vi "Dresden R2R Sputter 03.02.2018 IY24.vi"() -> ()   [LabVIEW 2009] (continued)
                                }
                                }
                                frame #1 {
                                n17381 = local read "Semi"() -> (w25829:bool)
                                n17382 = case shown="False" w25829 {
                                frame #0 {
                                n17383 = local write "Ch2_PV13"(TRUE ("P03")) -> ()
                                n17384 = Wait Until Next ms Multiple(millisecond multiple=u32 1000) -> ()  [unwired: 1 out]
                                }
                                frame #1 {
                                }
                                }
                                }
                                }
                              }
                              frame #1 {
                              }
                            }
                          }
                          frame #8 {
                            # "OPEN PC-BV"
                            n17385 = local read "Semi"() -> (w25832:bool)
                            n17386 = case shown="False" w25832 {
                              frame #0 {
                                n17387 = stacked-sequence {
                                frame #0 {
                                n17388 = local read "Semi"() -> (w25833:bool)
                                n17389 = case shown="False" w25833 {
                                frame #0 {
                                n17390 = stacked-sequence {
                                frame #0 {
                                n17391 = local read "Semi"() -> (w25834:bool)
                                n17392 = case shown="False" w25834 {
                                frame #0 {
                                n17393 = local write "Pc_bv2_auto_open"(TRUE ("Tp1_auto_start")) -> ()
                                }
                                frame #1 {
                                }
                                }
                                }
                                frame #1 {
                                n17394 = local read "Semi"() -> (w25836:bool)
                                n17395 = case shown="False" w25836 {
                                frame #0 {
                                n17396 = Wait (ms)(milliseconds to wait=u32 1000) -> ()  [unwired: 1 out]
                                }
                                frame #1 {
                                }
                                }
                                }
                                frame #2 {
                                n17397 = local read "Semi"() -> (w25838:bool)
                                n17398 = case shown="False" w25838 {
                                frame #0 {
                                n17399 = while {
                                i -> [w25844]
                                stop <- w25840 stop-if-true
                                n17400 = local read "Pc_bv_opened_ch2"() -> (w25842:bool)
                                n17401 = Greater?(x=w25844, y=120) -> (0:w25843:bool)
                                n17402 = local read "Semi"() -> (w25841:bool)
                                n17403 = Compound Arithmetic op=OR(w25841, w25842, w25843) -> (w25840:bool)
                                n17404 = Wait (ms)(milliseconds to wait=u32 500) -> ()  [unwired: 1 out]
                                }
                                }
                                frame #1 {
                                }
                                }
                                }
                                frame #3 {
                                n17405 = local read "Semi"() -> (w25846:bool)
                                n17406 = case shown="False" w25846 {
                                frame #0 {
                                n17407 = local read "Pc_bv_opened_ch2"() -> (w25847:bool)
                                n17408 = case shown="False" w25847 {
                                frame #0 {
                                n17409 = local write "Pc_bv2_auto_open"(TRUE ("Pc_bv1_auto_open")) -> ()
                                }
                                frame #1 {
                                }
                                }
                                }
                                frame #1 {
                                }
                                }
                                }
                                frame #4 {
                                n17410 = local read "Semi"() -> (w25849:bool)
                                n17411 = case shown="False" w25849 {
                                frame #0 {
                                n17412 = local read "Pc_bv_opened_ch2"() -> (w25850:bool)
                                n17413 = case shown="False" w25850 {
                                frame #0 {
                                n17414 = Wait (ms)(milliseconds to wait=u32 1000) -> ()  [unwired: 1 out]
                                }
                                frame #1 {
                                }
                                }
                                }
                                frame #1 {
                                }
                                }
                                }
                                frame #5 {
                                n17415 = local read "Semi"() -> (w25852:bool)
                                n17416 = case shown="False" w25852 {
                                frame #0 {
                                n17417 = while {
                                i -> [w25858]
                                stop <- w25854 stop-if-true
                                n17418 = local read "Pc_bv_opened_ch2"() -> (w25856:bool)
                                n17419 = Greater?(x=w25858, y=120) -> (0:w25857:bool)
                                n17420 = local read "Semi"() -> (w25855:bool)
                                n17421 = Compound Arithmetic op=OR(w25855, w25856, w25857) -> (w25854:bool)
                                n17422 = Wait (ms)(milliseconds to wait=u32 500) -> ()  [unwired: 1 out]
                                }
                                }
                                frame #1 {
                                }
                                }
                                }
                                frame #6 {
                                n17423 = local read "Semi"() -> (w25860:bool)
                                n17424 = case shown="False" w25860 {
                                frame #0 {
                                n17425 = local read "Pc_bv_opened_ch2"() -> (w25861:bool)
                                n17426 = case shown="False" w25861 {
                                frame #0 {
                                n17427 = local write "Error Message"("Start up process  cancelled\nbecause  PC-BV not opened.\nPlease check PC-BV2 connections." ("Error Message")) -> ()
                                n17428 = Wait (ms)(milliseconds to wait=u32 1000) -> ()  [unwired: 1 out]
                                }
                                frame #1 {
                                }
                                }
                                }
                                frame #1 {
                                }
                                }
                                }
                                }
                                }
                                frame #1 {
                                }
                                }
                                }
                                frame #1 {
                                n17429 = local read "Semi"() -> (w25864:bool)
                                n17430 = case shown="False" w25864 {
                                frame #0 {
                                n17431 = local write "Ch2_PV14"(TRUE ("P03")) -> ()
                                n17432 = Wait Until Next ms Multiple(millisecond multiple=u32 1000) -> ()  [unwired: 1 out]
                                }
                                frame #1 {
                                }
                                }
                                }
                                }
                              }
                              frame #1 {
                              }
                            }
                          }
                          frame #9 {
                            # "OPEN/CLOSE TRNS GV-BP2"
                            n17433 = local read "Semi"() -> (w25867:bool)
                            n17434 = case shown="False" w25867 {
                              frame #0 {
                                n17435 = stacked-sequence {
                                frame #0 {
                                n17436 = local read "Semi"() -> (w25868:bool)
                                n17437 = case shown="False" w25868 {
                                frame #0 {
                                n17438 = while {
                                i -> [w25877]
                                stop <- w25872 stop-if-true
                                n17439 = Greater?(x=w25877, y=50) -> (0:w25875:bool)
                                n17440 = case shown="True" w25875 {
                                frame #0 {
                                }
                                frame #1 {
                                n17441 = local read "Ch3_pressure"() -> (w25891:dbl)
                                n17442 = Less?(x=w25891, y=1) -> (x < y?=w25890:bool)
                                n17443 = case shown="True" w25890 {
                                frame #0 {
                                n17444 = local write "Error Message"("Start up process  cancelled\nbecause  Trns GV-BP2 not closed.\nPlease check \nTrns GV-BP2 connections." ("Error Message")) -> ()
                                }
                                frame #1 {
                                n17445 = local write "Error Message"("Start up process  cancelled\nbecause  Trns GV-BP2 not opened.\nPlease check \nTrns GV-BP2 connections." ("Error Message")) -> ()
                                }
                                }
                                n17446 = local write "Semi"(TRUE ("Semi")) -> ()
                                }
                                }
                                n17447 = local read "Ch3_pressure"() -> (w25871:dbl)
                                n17448 = Less?(x=w25871, y=1) -> (x < y?=w25869:bool)
                                n17449 = case shown="False" w25869 {
                                tunnel: [w25879 w25885] -> w25874
                                frame #0 {
                                n17450 = local read "Ch2_trns_gv_bp2_di"() -> (w25878:bool)
                                n17451 = case shown="True" w25878 {
                                tunnel: [TRUE FALSE] -> w25879
                                frame #0 {
                                }
                                frame #1 {
                                n17452 = local write "Ch2_trns_gv_bp2_do"(FALSE ("Ch1_Tp_bv_do")) -> ()
                                n17453 = Wait Until Next ms Multiple(millisecond multiple=u32 200) -> ()  [unwired: 1 out]
                                }
                                }
                                }
                                frame #1 {
                                n17454 = local read "Ch2_trns_gv_bp2_di"() -> (w25884:bool)
                                n17455 = case shown="False" w25884 {
                                tunnel: [FALSE TRUE] -> w25885
                                frame #0 {
                                n17456 = local write "Ch2_trns_gv_bp2_do"(TRUE ("Ch1_Tp_bv_do")) -> ()
                                n17457 = Wait Until Next ms Multiple(millisecond multiple=u32 200) -> ()  [unwired: 1 out]
                                }
                                frame #1 {
                                }
                                }
                                }
                                }
                                n17458 = local read "Semi"() -> (w25873:bool)
                                n17459 = Or(x=w25874, y=w25873) -> (x .or. y?=w25872:bool)
                                }
                                }
                                frame #1 {
                                }
                                }
                                }
                                frame #1 {
                                n17460 = local read "Semi"() -> (w25896:bool)
                                n17461 = case shown="False" w25896 {
                                frame #0 {
                                n17462 = local write "Ch2_PV15"(TRUE ("P03")) -> ()
                                n17463 = Wait Until Next ms Multiple(millisecond multiple=u32 1000) -> ()  [unwired: 1 out]
                                }
                                frame #1 {
                                }
                                }
                                }
                                }
                              }
                              frame #1 {
                              }
                            }
                          }
                          frame #10 {
                            # "OPEN/CLOSE TRNS GV-BP"
                            n17464 = local read "Semi"() -> (w25899:bool)
                            n17465 = case shown="False" w25899 {
                              frame #0 {
                                n17466 = stacked-sequence {
                                frame #0 {
                                n17467 = local read "Semi"() -> (w25900:bool)
                                n17468 = case shown="False" w25900 {
                                frame #0 {
                                n17469 = while {
                                i -> [w25909]
                                stop <- w25904 stop-if-true
                                n17470 = Greater?(x=w25909, y=50) -> (0:w25907:bool)
                                n17471 = case shown="True" w25907 {
                                frame #0 {
                                }
                                frame #1 {
                                n17472 = local read "Ch1_pressure"() -> (w25923:dbl)
                                n17473 = Less?(x=w25923, y=1) -> (x < y?=w25922:bool)
                                n17474 = case shown="True" w25922 {
                                frame #0 {
                                n17475 = local write "Error Message"("Start up process  cancelled\nbecause  Trns GV-BP2 not closed.\nPlease check \nTrns GV-BP2 connections." ("Error Message")) -> ()
                                }
                                frame #1 {
                                n17476 = local write "Error Message"("Start up process  cancelled\nbecause  Trns GV-BP not opened.\nPlease check \nTrns GV-BP connections." ("Error Message")) -> ()
                                }
                                }
                                n17477 = local write "Semi"(TRUE ("Semi")) -> ()
                                }
                                }
                                n17478 = local read "Ch1_pressure"() -> (w25903:dbl)
                                n17479 = Less?(x=w25903, y=1) -> (x < y?=w25901:bool)
                                n17480 = case shown="True" w25901 {
                                tunnel: [w25911 w25917] -> w25906
                                frame #0 {
                                n17481 = local read "Ch2_trns_gv_bp_di"() -> (w25910:bool)
                                n17482 = case shown="True" w25910 {
                                tunnel: [TRUE FALSE] -> w25911
                                frame #0 {
                                }
                                frame #1 {
                                n17483 = local write "Ch2_trns_gv_bp_do"(FALSE ("Ch1_Tp_bv_do")) -> ()
                                n17484 = Wait Until Next ms Multiple(millisecond multiple=u32 200) -> ()  [unwired: 1 out]
                                }
                                }
                                }
                                frame #1 {
                                n17485 = local read "Ch2_trns_gv_bp_di"() -> (w25916:bool)
                                n17486 = case shown="False" w25916 {
                                tunnel: [FALSE TRUE] -> w25917
                                frame #0 {
                                n17487 = local write "Ch2_trns_gv_bp_do"(TRUE ("Ch1_Tp_bv_do")) -> ()
                                n17488 = Wait Until Next ms Multiple(millisecond multiple=u32 200) -> ()  [unwired: 1 out]
                                }
                                frame #1 {
                                }
                                }
                                }
                                }
                                n17489 = local read "Semi"() -> (w25905:bool)
                                n17490 = Or(x=w25906, y=w25905) -> (x .or. y?=w25904:bool)
                                }
                                }
                                frame #1 {
                                }
                                }
                                }
                                frame #1 {
                                n17491 = local read "Semi"() -> (w25928:bool)
                                n17492 = case shown="False" w25928 {
                                frame #0 {
                                n17493 = local write "Ch2_PV16"(TRUE ("P03")) -> ()
                                n17494 = Wait Until Next ms Multiple(millisecond multiple=u32 1000) -> ()  [unwired: 1 out]
                                }
                                frame #1 {
                                }
                                }
                                }
                                }
                              }
                              frame #1 {
                              }
                            }
                          }
                          frame #11 {
                            # "CHECK CH-PRESSURE"
                            n17495 = local read "Semi"() -> (w25931:bool)
                            n17496 = case shown="False" w25931 {
                              frame #0 {
                                n17497 = stacked-sequence {
                                frame #0 {
                                n17498 = local read "Semi"() -> (w25932:bool)
                                n17499 = case shown="False" w25932 {
                                frame #0 {
                                n17500 = while {
                                i -> [w25941]
                                stop <- w25936 stop-if-true
                                n17501 = Greater?(x=w25941, y=600) -> (0:w25939:bool)
                                n17502 = case shown="True" w25939 {
                                frame #0 {
                                }
                                frame #1 {
                                n17503 = local write "Semi"(TRUE ("Semi")) -> ()
                                n17504 = local write "Error Message"("Start up process was cancelled.\nPlease check chamber \nvacuum connections." ("Error Message")) -> ()
                                }
                                }
                                n17505 = local read "Ch2_pressure"() -> (w25935:dbl)
                                n17506 = Less?(x=w25935, y=0.9) -> (x < y?=w25933:bool)
                                n17507 = case shown="False" w25933 {
                                tunnel: [FALSE TRUE] -> w25938
                                frame #0 {
                                n17508 = Wait Until Next ms Multiple(millisecond multiple=u32 500) -> ()  [unwired: 1 out]
                                }
                                frame #1 {
                                }
                                }
                                n17509 = local read "Semi"() -> (w25937:bool)
                                n17510 = Or(x=w25938, y=w25937) -> (x .or. y?=w25936:bool)
                                }
                                }
                                frame #1 {
                                }
                                }
                                }
                                frame #1 {
                                n17511 = local read "Semi"() -> (w25947:bool)
                                n17512 = case shown="False" w25947 {
                                frame #0 {
                                n17513 = local write "Ch2_PV17"(TRUE ("P03")) -> ()
                                n17514 = Wait Until Next ms Multiple(millisecond multiple=u32 1000) -> ()  [unwired: 1 out]
                                }
                                frame #1 {
                                }
                                }
                                }
                                }
                              }
                              frame #1 {
                              }
                            }
                          }
                          frame #12 {
                            # "OPEN BG-BV"
                            n17515 = local read "Semi"() -> (w25950:bool)
                            n17516 = case shown="False" w25950 {
                              frame #0 {
                                n17517 = stacked-sequence {
                                frame #0 {
                                n17518 = local read "Semi"() -> (w25951:bool)
                                n17519 = case shown="False" w25951 {
                                frame #0 {
                                n17520 = while {
                                i -> [w25958]
                                stop <- w25953 stop-if-true
                                n17521 = Greater?(x=w25958, y=50) -> (0:w25956:bool)
                                n17522 = case shown="True" w25956 {
                                frame #0 {
                                }
                                frame #1 {
                                n17523 = local write "Semi"(TRUE ("Semi")) -> ()
                                n17524 = local write "Error Message"("Start up process  cancelled\nbecause  BG-BV not opened.\nPlease check BG-BV2 connections." ("Error Message")) -> ()
                                }
                                }
                                n17525 = local read "Ch2_Bg_bv_di"() -> (w25952:bool)
                                n17526 = case shown="False" w25952 {
                                tunnel: [FALSE TRUE] -> w25955
                                frame #0 {
                                n17527 = Wait Until Next ms Multiple(millisecond multiple=u32 200) -> ()  [unwired: 1 out]
                                n17528 = local write "Ch2_Bg_bv_do"(TRUE ("Ch1_Tp_bv_do")) -> ()
                                }
                                frame #1 {
                                }
                                }
                                n17529 = local read "Semi"() -> (w25954:bool)
                                n17530 = Or(x=w25955, y=w25954) -> (x .or. y?=w25953:bool)
                                }
                                }
                                frame #1 {
                                }
                                }
                                }
                                frame #1 {
                                n17531 = local read "Semi"() -> (w25965:bool)
                                n17532 = case shown="False" w25965 {
                                frame #0 {
                                n17533 = local write "Ch2_PV18"(TRUE ("P03")) -> ()
                                n17534 = Wait Until Next ms Multiple(millisecond multiple=u32 1000) -> ()  [unwired: 1 out]
                                }
                                frame #1 {
                                }
                                }
                                }
                                }
                              }
                              frame #1 {
                              }
                            }
                          }
                          frame #13 {
                            # "CHECK CH-PRESSURE"
                            n17535 = local read "Semi"() -> (w25968:bool)
                            n17536 = case shown="False" w25968 {
                              frame #0 {
                                n17537 = stacked-sequence {
                                frame #0 {
                                n17538 = local read "Semi"() -> (w25969:bool)
                                n17539 = case shown="False" w25969 {
                                frame #0 {
                                n17540 = while {
                                i -> [w25978]
                                stop <- w25973 stop-if-true
                                n17541 = Greater?(x=w25978, y=240) -> (0:w25976:bool)
                                n17542 = case shown="True" w25976 {
                                frame #0 {
                                }
                                frame #1 {
                                n17543 = local write "Semi"(TRUE ("Semi")) -> ()
                                n17544 = local write "Error Message"("Start up process was cancelled.\nPlease check chamber \nvacuum connections." ("Error Message")) -> ()
                                }
                                }
                                n17545 = local read "Ch2_pressure"() -> (w25972:dbl)
                                n17546 = Less?(x=w25972, y=0.9) -> (x < y?=w25970:bool)
                                n17547 = case shown="False" w25970 {
                                tunnel: [FALSE TRUE] -> w25975
                                frame #0 {
                                n17548 = Wait Until Next ms Multiple(millisecond multiple=u32 500) -> ()  [unwired: 1 out]
                                }
                                frame #1 {
                                }
                                }
                                n17549 = local read "Semi"() -> (w25974:bool)
                                n17550 = Or(x=w25975, y=w25974) -> (x .or. y?=w25973:bool)
                                }
                                }
                                frame #1 {
                                }
                                }
                                }
                                frame #1 {
                                n17551 = local read "Semi"() -> (w25984:bool)
                                n17552 = case shown="False" w25984 {
                                frame #0 {
                                n17553 = local write "Ch2_PV19"(TRUE ("P03")) -> ()
                                n17554 = Wait Until Next ms Multiple(millisecond multiple=u32 1000) -> ()  [unwired: 1 out]
                                }
                                frame #1 {
                                }
                                }
                                }
                                }
                              }
                              frame #1 {
                              }
                            }
                          }
                          frame #14 {
                            # "START TP"
                            n17555 = local read "Semi"() -> (w25987:bool)
                            n17556 = case shown="False" w25987 {
                              frame #0 {
                                n17557 = stacked-sequence {
                                frame #0 {
                                n17558 = local read "Semi"() -> (w25988:bool)
                                n17559 = case shown="False" w25988 {
                                frame #0 {
                                n17560 = stacked-sequence {
                                frame #0 {
                                n17561 = local read "Semi"() -> (w25989:bool)
                                n17562 = case shown="False" w25989 {
                                frame #0 {
                                n17563 = local write "Tp2_auto_start"(TRUE ("Tp1_auto_start")) -> ()
                                }
                                frame #1 {
                                }
                                }
                                }
                                frame #1 {
                                n17564 = local read "Semi"() -> (w25991:bool)
                                n17565 = case shown="False" w25991 {
                                frame #0 {
                                n17566 = Wait (ms)(milliseconds to wait=u32 1000) -> ()  [unwired: 1 out]
                                }
                                frame #1 {
                                }
                                }
                                }
                                frame #2 {
                                n17567 = local read "Semi"() -> (w25993:bool)
                                n17568 = case shown="False" w25993 {
                                frame #0 {
                                n17569 = while {
                                i -> [w25999]
                                stop <- w25995 stop-if-true
                                n17570 = local read "TP2_working"() -> (w25997:bool)
                                n17571 = Greater?(x=w25999, y=120) -> (0:w25998:bool)
                                n17572 = local read "Semi"() -> (w25996:bool)
                                n17573 = Compound Arithmetic op=OR(w25996, w25997, w25998) -> (w25995:bool)
                                n17574 = Wait (ms)(milliseconds to wait=u32 500) -> ()  [unwired: 1 out]
                                }
                                }
                                frame #1 {
                                }
                                }
                                }
                                frame #3 {
                                n17575 = local read "Semi"() -> (w26001:bool)
                                n17576 = case shown="False" w26001 {
                                frame #0 {
                                n17577 = local read "TP2_working"() -> (w26002:bool)
                                n17578 = case shown="False" w26002 {
                                frame #0 {
                                n17579 = local write "Tp2_auto_start"(TRUE ("Pc_bv1_auto_open")) -> ()
                                }
                                frame #1 {
                                }
                                }
                                }
                                frame #1 {
                                }
                                }
                                }
                                frame #4 {
                                n17580 = local read "Semi"() -> (w26004:bool)
                                n17581 = case shown="False" w26004 {
                                frame #0 {
                                n17582 = local read "TP2_working"() -> (w26005:bool)
                                n17583 = case shown="False" w26005 {
                                frame #0 {
                                n17584 = Wait (ms)(milliseconds to wait=u32 1000) -> ()  [unwired: 1 out]
                                }
                                frame #1 {
                                }
                                }
                                }
                                frame #1 {
                                }
                                }
                                }
                                frame #5 {
                                n17585 = local read "Semi"() -> (w26007:bool)
                                n17586 = case shown="False" w26007 {
                                frame #0 {
                                n17587 = while {
                                i -> [w26013]
                                stop <- w26009 stop-if-true
                                n17588 = local read "TP2_working"() -> (w26011:bool)
                                n17589 = Greater?(x=w26013, y=120) -> (0:w26012:bool)
                                n17590 = local read "Semi"() -> (w26010:bool)
                                n17591 = Compound Arithmetic op=OR(w26010, w26011, w26012) -> (w26009:bool)
                                n17592 = Wait (ms)(milliseconds to wait=u32 500) -> ()  [unwired: 1 out]
                                }
                                }
                                frame #1 {
                                }
                                }
                                }
                                frame #6 {
                                n17593 = local read "Semi"() -> (w26015:bool)
                                n17594 = case shown="False" w26015 {
                                frame #0 {
                                n17595 = local read "TP2_working"() -> (w26016:bool)
                                n17596 = case shown="False" w26016 {
                                frame #0 {
                                n17597 = local write "Error Message"("Start up process  cancelled\nbecause  TP not started.\nPlease check TP2 connections." ("Error Message")) -> ()
                                n17598 = Wait (ms)(milliseconds to wait=u32 1000) -> ()  [unwired: 1 out]
                                }
                                frame #1 {
                                }
                                }
                                }
                                frame #1 {
                                }
                                }
                                }
                                }
                                }
                                frame #1 {
                                }
                                }
                                }
                                frame #1 {
                                n17599 = local read "Semi"() -> (w26019:bool)
                                n17600 = case shown="False" w26019 {
                                frame #0 {
                                n17601 = local write "Ch2_PV20"(TRUE ("P03")) -> ()
                                n17602 = Wait Until Next ms Multiple(millisecond multiple=u32 1000) -> ()  [unwired: 1 out]
                                }
                                frame #1 {
                                }
                                }
                                }
                                }
                              }
                              frame #1 {
                              }
                            }
                          }
                        }
                      }
                      frame #1 {
                      }
                    }
                  }
                  frame #1 {
                    # "PUMPING CH2 HIGHER THAN 0.9 TORR"
                    n17603 = local read "Semi"() -> (w26022:bool)
                    n17604 = case shown="False" w26022 {
                      frame #0 {
                        n17605 = stacked-sequence {
                          frame #0 {
                            # "STOP TP"
                            n17606 = local read "Semi"() -> (w26023:bool)
                            n17607 = case shown="False" w26023 {
                              frame #0 {
                                n17608 = stacked-sequence {
                                frame #0 {
                                n17609 = local read "Semi"() -> (w26024:bool)
                                n17610 = case shown="False" w26024 {
                                frame #0 {
                                n17611 = stacked-sequence {
                                frame #0 {
                                n17612 = local read "Semi"() -> (w26025:bool)
                                n17613 = case shown="False" w26025 {
                                frame #0 {
                                n17614 = local write "Tp2_auto_stop"(TRUE ("Tp1_auto_start")) -> ()
                                }
                                frame #1 {
                                }
                                }
                                }
                                frame #1 {
                                n17615 = local read "Semi"() -> (w26027:bool)
                                n17616 = case shown="False" w26027 {
                                frame #0 {
                                n17617 = Wait (ms)(milliseconds to wait=u32 1000) -> ()  [unwired: 1 out]
                                }
                                frame #1 {
                                }
                                }
                                }
                                frame #2 {
                                n17618 = local read "Semi"() -> (w26029:bool)
                                n17619 = case shown="False" w26029 {
                                frame #0 {
                                n17620 = while {
                                i -> [w26035]
                                stop <- w26031 stop-if-true
                                n17621 = local read "Tp2_stopped"() -> (w26033:bool)
                                n17622 = Greater?(x=w26035, y=120) -> (0:w26034:bool)
                                n17623 = local read "Semi"() -> (w26032:bool)
                                n17624 = Compound Arithmetic op=OR(w26032, w26033, w26034) -> (w26031:bool)
                                n17625 = Wait (ms)(milliseconds to wait=u32 500) -> ()  [unwired: 1 out]
                                }
                                }
                                frame #1 {
                                }
                                }
                                }
                                frame #3 {
                                n17626 = local read "Semi"() -> (w26037:bool)
                                n17627 = case shown="False" w26037 {
                                frame #0 {
                                n17628 = local read "Tp2_stopped"() -> (w26038:bool)
                                n17629 = case shown="False" w26038 {
                                frame #0 {
                                n17630 = local write "Tp2_auto_stop"(TRUE ("Pc_bv1_auto_open")) -> ()
                                }
                                frame #1 {
                                }
                                }
                                }
                                frame #1 {
                                }
                                }
                                }
                                frame #4 {
                                n17631 = local read "Semi"() -> (w26040:bool)
                                n17632 = case shown="False" w26040 {
                                frame #0 {
                                n17633 = local read "Tp2_stopped"() -> (w26041:bool)
                                n17634 = case shown="False" w26041 {
                                frame #0 {
                                n17635 = Wait (ms)(milliseconds to wait=u32 1000) -> ()  [unwired: 1 out]
                                }
                                frame #1 {
                                }
                                }
                                }
                                frame #1 {
                                }
                                }
                                }
                                frame #5 {
                                n17636 = local read "Semi"() -> (w26043:bool)
                                n17637 = case shown="False" w26043 {
                                frame #0 {
                                n17638 = while {
                                i -> [w26049]
                                stop <- w26045 stop-if-true
                                n17639 = local read "Tp2_stopped"() -> (w26047:bool)
                                n17640 = Greater?(x=w26049, y=120) -> (0:w26048:bool)
                                n17641 = local read "Semi"() -> (w26046:bool)
                                n17642 = Compound Arithmetic op=OR(w26046, w26047, w26048) -> (w26045:bool)
                                n17643 = Wait (ms)(milliseconds to wait=u32 500) -> ()  [unwired: 1 out]
                                }
                                }
                                frame #1 {
                                }
                                }
                                }
                                frame #6 {
                                n17644 = local read "Semi"() -> (w26051:bool)
                                n17645 = case shown="False" w26051 {
                                frame #0 {
                                n17646 = local read "Tp2_stopped"() -> (w26052:bool)
                                n17647 = case shown="False" w26052 {
                                frame #0 {
                                n17648 = local write "Error Message"("Start up process  cancelled\nbecause  TP2 not stopped.\nPlease check TP2 connections." ("Error Message")) -> ()
                                n17649 = Wait (ms)(milliseconds to wait=u32 1000) -> ()  [unwired: 1 out]
                                }
                                frame #1 {
                                }
                                }
                                }
                                frame #1 {
                                }
                                }
                                }
                                }
                                }
                                frame #1 {
                                }
                                }
                                }
                                frame #1 {
                                n17650 = local read "Semi"() -> (w26055:bool)
                                n17651 = case shown="False" w26055 {
                                frame #0 {
                                n17652 = local write "Ch2_PA6"(TRUE ("PA2")) -> ()
                                n17653 = Wait Until Next ms Multiple(millisecond multiple=u32 1000) -> ()  [unwired: 1 out]
                                }
                                frame #1 {
                                }
                                }
                                }
                                }
                              }
                              frame #1 {
                              }
                            }
                          }
                          frame #1 {
                            # "CLOSE CH-CC"
                            n17654 = local read "Semi"() -> (w26058:bool)
                            n17655 = case shown="False" w26058 {
                              frame #0 {
                                n17656 = stacked-sequence {
                                frame #0 {
                                n17657 = local read "Semi"() -> (w26059:bool)
                                n17658 = case shown="False" w26059 {
                                frame #0 {
                                n17659 = while {
                                i -> [w26066]
                                stop <- w26060 stop-if-true
                                n17660 = Greater?(x=w26066, y=50) -> (0:w26064:bool)
                                n17661 = case shown="True" w26064 {
                                frame #0 {
                                }
                                frame #1 {
                                n17662 = local write "Semi"(TRUE ("Semi")) -> ()
                                n17663 = local write "Error Message"("Start up process  cancelled\nbecause  CH2-CC not closed.\nPlease check  CH2-CC connections." ("Error Message")) -> ()
                                }
                                }
                                n17664 = local read "Ch2_Cc_on_off_di"() -> (w26063:bool)
                                n17665 = case shown="True" w26063 {
                                tunnel: [TRUE FALSE] -> w26062
                                frame #0 {
                                }
                                frame #1 {
                                n17666 = Wait Until Next ms Multiple(millisecond multiple=u32 200) -> ()  [unwired: 1 out]
                                n17667 = local write "Ch2_Cc_on_off_do"(FALSE ("Ch1_Tp_bv_do")) -> ()